vi "VP_RT_standard.vi"() -> ()   [LabVIEW 2015] (continued)
      }
      frame True {
        n40 = shared-variable ".\\Interloop communication.lvlib\\System command"(Command_Enum."Stop System" ("System command")) -> (error out=w66:errorcluster)  [unwired: 1 in]
        n41 = shared-variable ".\\Interloop communication.lvlib\\New Command"(TRUE ("New Command"), error in=w66) -> ()  [unwired: 1 out]
      }
    }
    n42 = Wait Until Next ms Multiple(millisecond multiple=u32 100) -> ()  [unwired: 1 out]
    "Command Loop Iterations" <- w20
  }
  n43 = timed-loop {
    timing: w9 -> [_]
    timing-out: [_] -> w8
    shift-right: [w74] -> _
    shift-left: w4 -> [w71]
    shift-right: [w83] -> _
    shift-left: w2 -> [w75]
    shift-right: [w82] -> _
    shift-left: w1 -> [w76]
    shift-right: [w78] -> _
    shift-left: w3 -> [w79]
    i -> [w80]
    stop <- w85 stop-if-true
    # "Main Loop"
    n44 = node-c288() -> ()  [unwired: 1 in, 1 out]
    n45 = local read "Snake Scan Reference FPGA or EPICS"() -> (w73:enum16{"FPGA Snake Scan", "EPICS Snake Scan"})
    n46 = Format Into String(format string="%s", w71) -> (resulting string=w70:string)  [unwired: 2 in, 1 out]
    n47 = shared-variable "RT CompactRIO Target\\RT_EPICS_Shared_Variables.lvlib\\2iddVELO:VP:RT_State"(w70) -> ()  [unwired: 1 in, 1 out]
    n48 = case shown="\"End Scan\"" w71 {
      tunnel: [w92 w102 w185 w272 w308 w423 w456 w469 w492 w533 w554 w624 w639 w651] -> w84
      tunnel: [FALSE ("Stop") FALSE ("Stop") FALSE ("Stop") FALSE ("Stop") FALSE ("Stop") FALSE ("Stop") FALSE ("Stop") FALSE ("Stop") _ FALSE ("Stop") FALSE ("Stop") FALSE ("Stop") FALSE ("Stop") TRUE ("Stop")] -> w85
      tunnel: [w95 w116 w184 w274 w306 w422 w455 w471 w483 w516 w580 w619 w634 w648] -> w83
      tunnel: [w87 w110 w183 w268 w305 w421 w454 w462 w482 w520 w578 w622 w633 w653] -> w82
      tunnel: w76 -> [w93 w113 w187 w269 w315 w425 w457 w472 w490 w518 w595 w614 w637 w657]
      tunnel: w75 -> [w94 w116 w186 w274 w316 w426 w458 w473 w491 w517 w581 w616 w643 w658]
      tunnel: w79 -> [w92 w102 w185 _ w308 w423 w456 w469 w492 w533 w555 w624 w639 _]
      tunnel: [i64 0 i64 0 i64 0 i64 50 i64 0 i64 0 i64 0 i64 0 i64 0 i64 250 w534 i64 0 i64 0 i64 0] -> w77
      tunnel: w73 -> [_ _ _ _ w302 w418 _ _ _ _ _ _ _ _]
      frame "Initialization", Default {
        n49 = xnode "Invoke Method"("FPGA VI Reference In"=w94, "error in"=w93, "Requested Depth"="Requested Depth") -> ("FPGA VI Reference Out"=w97:refnum<k20>, "error out"=w96:errorcluster, "Actual Depth"=→"Actual Depth":u32)
        n50 = xnode "Read/Write Control"("FPGA VI Reference In"=w97, "error in"=w96, "Datalog Time Period (uSec)"="Datalog Time Period (uSec)", "Datalog Cases"="Datalog Cases") -> ("FPGA VI Reference Out"=w89:refnum<k20>, "error out"=w88:errorcluster)
        n51 = xnode "Read/Write Control"("FPGA VI Reference In"=w89, "error in"=w88) -> ("FPGA VI Reference Out"=w95:refnum<k20>, "error out"=w87:errorcluster, "Wait error"=w86:errorcluster)
        "FPGA wait error" <- w86
        n52 = shared-variable ".\\Interloop communication.lvlib\\FPGA startup error"(w86) -> ()  [unwired: 1 in, 1 out]
      }
      frame "Import Controller coeffs" {
        n53 = call "Read_coeff.vi"("error in (no error)"=w113, "sos gain SF controller file path"="file path sos gain SF Controller_xz1", "sos coeff file path"="file path soscoeff_xz1") -> ("b02(2)"=→"b02(2) xz1c":fxp<+/-,64,9>[], "b01(2)"=→"b01(2) xz1c":fxp<+/-,64,9>[], "-a02(2)"=→"-a02(2) xz1c":fxp<+/-,64,9>[], "-a01(2)"=→"-a01(2) xz1c":fxp<+/-,64,9>[], "error out"=w112:errorcluster, "sos gain SF Controller"=→"sos gain SF Controller xz1c":fxp<+/-,42,9>)  [unwired: 3 in]
        n54 = call "Read_coeff.vi"("error in (no error)"=w113, "sos gain SF controller file path"="file path sos gain SF Controller_xx1", "sos coeff file path"="file path soscoeff_xx1") -> ("b02(2)"=→"b02(2) xx1c":fxp<+/-,64,9>[], "b01(2)"=→"b01(2) xx1c":fxp<+/-,64,9>[], "-a02(2)"=→"-a02(2) xx1c":fxp<+/-,64,9>[], "-a01(2)"=→"-a01(2) xx1c":fxp<+/-,64,9>[], "error out"=w105:errorcluster, "sos gain SF Controller"=→"sos gain SF Controller xx1c":fxp<+/-,42,9>)  [unwired: 3 in]
        n55 = call "Read_coeff.vi"("error in (no error)"=w113, "sos gain SF controller file path"="file path sos gain SF Controller_xy1", "sos coeff file path"="file path soscoeff_xy1") -> ("b02(2)"=→"b02(2) xy1c":fxp<+/-,64,9>[], "b01(2)"=→"b01(2) xy1c":fxp<+/-,64,9>[], "-a02(2)"=→"-a02(2) xy1c":fxp<+/-,64,9>[], "-a01(2)"=→"-a01(2) xy1c":fxp<+/-,64,9>[], "error out"=w108:errorcluster, "sos gain SF Controller"=→"sos gain SF Controller xy1c":fxp<+/-,42,9>)  [unwired: 3 in]
        n56 = call "Read_coeff.vi"("error in (no error)"=w112, "sos gain SF controller file path"="file path sos gain SF Controller_yz1", "sos coeff file path"="file path soscoeff_yz1") -> ("b02(2)"=→"b02(2) yz1c":fxp<+/-,64,9>[], "b01(2)"=→"b01(2) yz1c":fxp<+/-,64,9>[], "-a02(2)"=→"-a02(2) yz1c":fxp<+/-,64,9>[], "-a01(2)"=→"-a01(2) yz1c":fxp<+/-,64,9>[], "error out"=w111:errorcluster, "sos gain SF Controller"=→"sos gain SF Controller yz1c":fxp<+/-,42,9>)  [unwired: 3 in]
        n57 = call "Read_coeff.vi"("error in (no error)"=w108, "sos gain SF controller file path"="file path sos gain SF Controller_yy1", "sos coeff file path"="file path soscoeff_yy1") -> ("b02(2)"=→"b02(2) yy1c":fxp<+/-,64,9>[], "b01(2)"=→"b01(2) yy1c":fxp<+/-,64,9>[], "-a02(2)"=→"-a02(2) yy1c":fxp<+/-,64,9>[], "-a01(2)"=→"-a01(2) yy1c":fxp<+/-,64,9>[], "error out"=w107:errorcluster, "sos gain SF Controller"=→"sos gain SF Controller yy1c":fxp<+/-,42,9>)  [unwired: 3 in]
        n58 = call "Read_coeff.vi"("error in (no error)"=w105, "sos gain SF controller file path"="file path sos gain SF Controller_yx1", "sos coeff file path"="file path soscoeff_yx1") -> ("b02(2)"=→"b02(2) yx1c":fxp<+/-,64,9>[], "b01(2)"=→"b01(2) yx1c":fxp<+/-,64,9>[], "-a02(2)"=→"-a02(2) yx1c":fxp<+/-,64,9>[], "-a01(2)"=→"-a01(2) yx1c":fxp<+/-,64,9>[], "error out"=w104:errorcluster, "sos gain SF Controller"=→"sos gain SF Controller yx1c":fxp<+/-,42,9>)  [unwired: 3 in]
        n59 = call "Read_coeff.vi"("error in (no error)"=w111, "sos gain SF controller file path"="file path sos gain SF Controller_zz1", "sos coeff file path"="file path soscoeff_zz1") -> ("b02(2)"=→"b02(2) zz1c":fxp<+/-,64,9>[], "b01(2)"=→"b01(2) zz1c":fxp<+/-,64,9>[], "-a02(2)"=→"-a02(2) zz1c":fxp<+/-,64,9>[], "-a01(2)"=→"-a01(2) zz1c":fxp<+/-,64,9>[], "error out"=w109:errorcluster, "sos gain SF Controller"=→"sos gain SF Controller zz1c":fxp<+/-,42,9>)  [unwired: 3 in]
        n60 = call "Read_coeff.vi"("error in (no error)"=w104, "sos gain SF controller file path"="file path sos gain SF Controller_zx1", "sos coeff file path"="file path soscoeff_zx1") -> ("b02(2)"=→"b02(2) zx1c":fxp<+/-,64,9>[], "b01(2)"=→"b01(2) zx1c":fxp<+/-,64,9>[], "-a02(2)"=→"-a02(2) zx1c":fxp<+/-,64,9>[], "-a01(2)"=→"-a01(2) zx1c":fxp<+/-,64,9>[], "error out"=w103:errorcluster, "sos gain SF Controller"=→"sos gain SF Controller zx1c":fxp<+/-,42,9>)  [unwired: 3 in]
        n61 = call "Read_coeff.vi"("error in (no error)"=w107, "sos gain SF controller file path"="file path sos gain SF Controller_zy1", "sos coeff file path"="file path soscoeff_zy1") -> ("b02(2)"=→"b02(2) zy1c":fxp<+/-,64,9>[], "b01(2)"=→"b01(2) zy1c":fxp<+/-,64,9>[], "-a02(2)"=→"-a02(2) zy1c":fxp<+/-,64,9>[], "-a01(2)"=→"-a01(2) zy1c":fxp<+/-,64,9>[], "error out"=w106:errorcluster, "sos gain SF Controller"=→"sos gain SF Controller zy1c":fxp<+/-,42,9>)  [unwired: 3 in]
        n62 = Merge Errors(w113, w103, w106, w109) -> (w110:errorcluster)
        "Coeff file import error" <- w110
      }
      frame "Update Controller Info" {
        n63 = local read "sos gain SF Controller yy1c"() -> (w246:fxp<+/-,42,9>)
        n64 = local read "sos gain SF Controller yz1c"() -> (w195:fxp<+/-,42,9>)
        n65 = local read "sos gain SF Controller yx1c"() -> (w234:fxp<+/-,42,9>)
        n66 = local read "sos gain SF Controller xy1c"() -> (w220:fxp<+/-,42,9>)
        n67 = local read "sos gain SF Controller zy1c"() -> (w225:fxp<+/-,42,9>)
        n68 = local read "sos gain SF Controller xz1c"() -> (w209:fxp<+/-,42,9>)
        n69 = local read "sos gain SF Controller xx1c"() -> (w251:fxp<+/-,42,9>)
        n70 = local read "sos gain SF Controller zz1c"() -> (w244:fxp<+/-,42,9>)
        n71 = local read "sos gain SF Controller zx1c"() -> (w230:fxp<+/-,42,9>)
        n72 = local read "-a01(2) yy1c"() -> (w250:fxp<+/-,64,9>[])
        n73 = local read "-a02(2) yy1c"() -> (w249:fxp<+/-,64,9>[])
        n74 = local read "-a01(2) yz1c"() -> (w214:fxp<+/-,64,9>[])
        n75 = local read "-a02(2) yz1c"() -> (w215:fxp<+/-,64,9>[])
        n76 = local read "-a01(2) yx1c"() -> (w235:fxp<+/-,64,9>[])
        n77 = local read "-a02(2) yx1c"() -> (w231:fxp<+/-,64,9>[])
        n78 = local read "-a01(2) xy1c"() -> (w216:fxp<+/-,64,9>[])
        n79 = local read "-a02(2) xy1c"() -> (w217:fxp<+/-,64,9>[])
        n80 = local read "-a01(2) zy1c"() -> (w221:fxp<+/-,64,9>[])
        n81 = local read "-a02(2) zy1c"() -> (w222:fxp<+/-,64,9>[])
        n82 = local read "-a01(2) xz1c"() -> (w213:fxp<+/-,64,9>[])
        n83 = local read "-a02(2) xz1c"() -> (w212:fxp<+/-,64,9>[])
        n84 = local read "-a01(2) xx1c"() -> (w255:fxp<+/-,64,9>[])
        n85 = local read "-a02(2) xx1c"() -> (w254:fxp<+/-,64,9>[])
        n86 = local read "-a01(2) zz1c"() -> (w245:fxp<+/-,64,9>[])
        n87 = local read "-a02(2) zz1c"() -> (w241:fxp<+/-,64,9>[])
        n88 = local read "-a01(2) zx1c"() -> (w226:fxp<+/-,64,9>[])
        n89 = local read "-a02(2) zx1c"() -> (w227:fxp<+/-,64,9>[])
        n90 = local read "b01(2) yy1c"() -> (w248:fxp<+/-,64,9>[])
        n91 = local read "b02(2) yy1c"() -> (w247:fxp<+/-,64,9>[])
        n92 = local read "b01(2) yz1c"() -> (w189:fxp<+/-,64,9>[])
        n93 = local read "b02(2) yz1c"() -> (w188:fxp<+/-,64,9>[])
        n94 = local read "b01(2) yx1c"() -> (w232:fxp<+/-,64,9>[])
        n95 = local read "b02(2) yx1c"() -> (w233:fxp<+/-,64,9>[])
        n96 = local read "b01(2) xy1c"() -> (w218:fxp<+/-,64,9>[])
        n97 = local read "b02(2) xy1c"() -> (w219:fxp<+/-,64,9>[])
        n98 = local read "b01(2) zy1c"() -> (w223:fxp<+/-,64,9>[])
        n99 = local read "b02(2) zy1c"() -> (w224:fxp<+/-,64,9>[])
        n100 = local read "b01(2) xz1c"() -> (w211:fxp<+/-,64,9>[])
        n101 = local read "b02(2) xz1c"() -> (w210:fxp<+/-,64,9>[])
        n102 = local read "b01(2) xx1c"() -> (w253:fxp<+/-,64,9>[])
        n103 = local read "b02(2) xx1c"() -> (w252:fxp<+/-,64,9>[])
        n104 = local read "b01(2) zz1c"() -> (w242:fxp<+/-,64,9>[])
        n105 = local read "b02(2) zz1c"() -> (w243:fxp<+/-,64,9>[])
        n106 = local read "b01(2) zx1c"() -> (w228:fxp<+/-,64,9>[])
        n107 = local read "b02(2) zx1c"() -> (w229:fxp<+/-,64,9>[])
        n108 = Or(x="Optics Z Reset", y="Reset All") -> (x .or. y?=w208:bool)
        n109 = Or(x="Sample Z Reset", y="Reset All") -> (x .or. y?=w205:bool)
        n110 = Or(x="Optics X Reset", y="Reset All") -> (x .or. y?=w239:bool)
        n111 = Or(x="Optics Y Reset", y="Reset All") -> (x .or. y?=w237:bool)
        n112 = Or(x="Sample X Reset", y="Reset All") -> (x .or. y?=w207:bool)
        n113 = Or(x="Sample Y Reset", y="Reset All") -> (x .or. y?=w206:bool)
        n114 = xnode "Read/Write Control"("FPGA VI Reference In"=w186, "error in"=w187, "Wait timer (ms)"="FPGA Wait Timer (ms)", "Controller Time Period (uSec)"="Controller Time Period (uSec)", "Controller Output Time Period (uSec)"="Controller Output Time Period (uSec)", "System Loop Type"="System Loop Type", "Controller Output Upper Limit"="Controller Output Upper Limit", "Controller Output Lower Limit"="Controller Output Lower Limit", "X-Stage nm to V Scaling"="X-Stage nm to V Scaling", "X-Stage Scaling Direction"="X-Stage Scaling Direction", "Y-Stage nm to V Scaling"="Y-Stage nm to V Scaling", "Z-Stage nm to V Scaling"="Z-Stage nm to V Scaling", "Plant Output Time Period (uSec)"="Plant Output Time Period (uSec)", "Reset Optics X"=w239, "Reset Optics Y"=w237, "Reset Optics Z"=w208, "Reset Sample X"=w207, "Reset Sample Y"=w206, "Reset Sample Z"=w205, "Optics X Stage Resolution (nm)"="Optics X Stage Resolution (nm)", "Optics Y Stage Resolution (nm)"="Optics Y Stage Resolution (nm)", "Optics Z Stage Resolution (nm)"="Optics Z Stage Resolution (nm)", "Sample X Stage Resolution (nm)"="Sample X Stage Resolution (nm)", "Sample Y Stage Resolution (nm)"="Sample Y Stage Resolution (nm)", "Sample Z Stage Resolution (nm)"="Sample Z Stage Resolution (nm)", "Scaling mV to V"="Scaling mV to V", "-a01(2) xx1"=w255, "-a02(2) xx1"=w254, "b01(2) xx1"=w253, "b02(2) xx1"=w252, "sos gain SF Controller xx1"=w251, "-a01(2) yy1"=w250, "-a02(2) yy1"=w249, "b01(2) yy1"=w248, "b02(2) yy1"=w247, "sos gain SF Controller yy1"=w246, "-a01(2) zz1"=w245, "-a02(2) zz1"=w241, "b01(2) zz1"=w242, "b02(2) zz1"=w243, "sos gain SF Controller zz1"=w244, "-a01(2) yx1"=w235, "-a02(2) yx1"=w231, "b01(2) yx1"=w232, "b02(2) yx1"=w233, "sos gain SF Controller yx1"=w234, "-a01(2) zx1"=w226, "-a02(2) zx1"=w227, "b01(2) zx1"=w228, "b02(2) zx1"=w229, "sos gain SF Controller zx1"=w230, "-a01(2) xy1"=w216, "-a02(2) xy1"=w217, "b01(2) xy1"=w218, "b02(2) xy1"=w219, "sos gain SF Controller xy1"=w220, "-a01(2) zy1"=w221, "-a02(2) zy1"=w222, "b01(2) zy1"=w223, "b02(2) zy1"=w224, "sos gain SF Controller zy1"=w225, "-a01(2) xz1"=w213, "-a02(2) xz1"=w212, "b01(2) xz1"=w211, "b02(2) xz1"=w210, "sos gain SF Controller xz1"=w209, "-a01(2) yz1"=w214, "-a02(2) yz1"=w215, "b01(2) yz1"=w189, "b02(2) yz1"=w188, "sos gain SF Controller yz1"=w195, "Analog Input Time Period (uSec)"="Analog Input Time Period (uSec)", "Optics and or Sample Stage"="Optics and or Sample Stage", "Y-Stage Scaling Direction"="Y-Stage Scaling Direction", "Z-Stage Scaling Direction"="Z-Stage Scaling Direction") -> ("FPGA VI Reference Out"=w184:refnum<k20>, "error out"=w183:errorcluster)
      }
      frame "Wait" {
        n115 = shared-variable ".\\Interloop communication.lvlib\\New Command"() -> (w273:bool, error out=w271:errorcluster)  [unwired: 1 in]
        n116 = case shown="True" w273 {
          tunnel: [w276 w277] -> w272
          tunnel: w271 -> [_ w281]
          tunnel: w269 -> [w275 w279]
          tunnel: [w275 w278] -> w268
          frame False {
            w276 = T10[] [enum."Wait"] items=["Initialization", "Import Controller coeffs", "Update Controller Info", "Wait", "Update Reference Info", "Update Detector Trigger Info", "Update Datalog Info", "Check FPGA Status", "Pre-Scan", "Start Scan", "Scanning", "End Scan", "Restart FPGA", "Stop FPGA"]
          }
          frame True {
            n117 = shared-variable ".\\Interloop communication.lvlib\\System command"() -> (w280:T7)  [unwired: 1 in, 1 out]
            "Last Command Executed" <- w280
            n118 = case shown="\"Stop System\"" w280 {
              tunnel: [w285 w288 w291 w294 w297 w301] -> w277
              tunnel: w279 -> [w284 w287 w290 w293 w296 w300]
              tunnel: [w283 w286 w289 w292 w295 w299] -> w278
              frame "Re-Initialize ", Default {
                w285 = T10[] [enum."Initialization", enum."Import Controller coeffs", enum."Update Controller Info", enum."Wait"] items=["Initialization", "Import Controller coeffs", "Update Controller Info", "Wait", "Update Reference Info", "Update Detector Trigger Info", "Update Datalog Info", "Check FPGA Status", "Pre-Scan", "Start Scan", "Scanning", "End Scan", "Restart FPGA", "Stop FPGA"]
                n119 = call <vilib>:"Clear Errors.vi"("error in (no error)"=w284) -> ("error out"=w283:errorcluster)  [unwired: 5 in, 1 out]
              }
              frame "Update Scan Settings" {
                w288 = T10[] [enum."Update Reference Info", enum."Update Detector Trigger Info", enum."Update Datalog Info", enum."Wait"] items=["Initialization", "Import Controller coeffs", "Update Controller Info", "Wait", "Update Reference Info", "Update Detector Trigger Info", "Update Datalog Info", "Check FPGA Status", "Pre-Scan", "Start Scan", "Scanning", "End Scan", "Restart FPGA", "Stop FPGA"]
                n120 = call <vilib>:"Clear Errors.vi"("error in (no error)"=w287) -> ("error out"=w286:errorcluster)  [unwired: 5 in, 1 out]
              }
              frame "Scan" {
                w291 = T10[] [enum."Update Reference Info", enum."Update Detector Trigger Info", enum."Update Datalog Info", enum."Pre-Scan", enum."Start Scan", enum."Scanning", enum."End Scan", enum."Wait"] items=["Initialization", "Import Controller coeffs", "Update Controller Info", "Wait", "Update Reference Info", "Update Detector Trigger Info", "Update Datalog Info", "Check FPGA Status", "Pre-Scan", "Start Scan", "Scanning", "End Scan", "Restart FPGA", "Stop FPGA"]
                n121 = call <vilib>:"Clear Errors.vi"("error in (no error)"=w290) -> ("error out"=w289:errorcluster)  [unwired: 5 in, 1 out]
              }
              frame "Stop Scan" {
                w294 = T10[] [enum."End Scan", enum."Wait"] items=["Initialization", "Import Controller coeffs", "Update Controller Info", "Wait", "Update Reference Info", "Update Detector Trigger Info", "Update Datalog Info", "Check FPGA Status", "Pre-Scan", "Start Scan", "Scanning", "End Scan", "Restart FPGA", "Stop FPGA"]
                n122 = call <vilib>:"Clear Errors.vi"("error in (no error)"=w293) -> ("error out"=w292:errorcluster)  [unwired: 5 in, 1 out]
              }
              frame "Restart FPGA" {
                w297 = T10[] [enum."Restart FPGA", enum."Initialization", enum."Import Controller coeffs", enum."Update Controller Info", enum."Wait"] items=["Initialization", "Import Controller coeffs", "Update Controller Info", "Wait", "Update Reference Info", "Update Detector Trigger Info", "Update Datalog Info", "Check FPGA Status", "Pre-Scan", "Start Scan", "Scanning", "End Scan", "Restart FPGA", "Stop FPGA"]
                n123 = call <vilib>:"Clear Errors.vi"("error in (no error)"=w296) -> ("error out"=w295:errorcluster)  [unwired: 5 in, 1 out]
              }
              frame "Stop System" {
                w301 = T10[] [enum."Stop FPGA"] items=["Initialization", "Import Controller coeffs", "Update Controller Info", "Wait", "Update Reference Info", "Update Detector Trigger Info", "Update Datalog Info", "Check FPGA Status", "Pre-Scan", "Start Scan", "Scanning", "End Scan", "Restart FPGA", "Stop FPGA"]
                n124 = call <vilib>:"Clear Errors.vi"("error in (no error)"=w300) -> ("error out"=w299:errorcluster)  [unwired: 5 in, 1 out]
                n125 = local write "Stop System (Careful!!)"(TRUE ("Stop")) -> ()
              }
            }
            n126 = shared-variable ".\\Interloop communication.lvlib\\New Command"(FALSE ("New Command"), error in=w281) -> ()  [unwired: 1 out]
          }
        }
      }
      frame "Update Reference Info" {
        w368 = errorcluster {"status"=FALSE, "code"=0, "source"=""}  # error in (no error)
        w371 = errorcluster {"status"=FALSE, "code"=0, "source"=""}  # error in (no error)
        w385 = errorcluster {"status"=FALSE, "code"=0, "source"=""}  # error in (no error)
        w364 = 40000000.0  # FPGA clock rate (Hz)
        n127 = local read "Measured Z Reference Time Period (Ticks)"() -> (w307:u32)
        n128 = case shown="\"EPICS Snake Scan\"" w302 {
          tunnel: ["X Ramp Start (nm)" w401] -> w323
          tunnel: ["X Ramp End (nm)" w400] -> w322
          tunnel: ["Y Ramp Start (nm)" w399] -> w321
          tunnel: ["Y Ramp End (nm)" w398] -> w320
          tunnel: ["Y Step Size (nm)" w402] -> w319
          tunnel: ["X Step Size (nm)" w405] -> w318
          tunnel: [w393 w403] -> w317
          tunnel: ["Y Step Size (nm)" w402] -> w314
          tunnel: ["X Ramp Start (nm)" w401] -> w313
          tunnel: ["X Ramp End (nm)" w400] -> w312
          tunnel: ["Y Ramp Start (nm)" w399] -> w311
          tunnel: ["Y Ramp End (nm)" w398] -> w310
          frame "FPGA Snake Scan", Default {
            n129 = local read "DT Frequency (Hz)"() -> (w393:dbl)
          }
          frame "EPICS Snake Scan" {
            w404 = fxp<+/-,16,16> 0.0 ("fixed-point type")
            n130 = shared-variable "RT CompactRIO Target\\RT_EPICS_Shared_Variables.lvlib\\2iddVELO:VP:Trigger_Freq_Hz"() -> (w403:dbl)  [unwired: 1 in, 1 out]
            "2iddVELO:VP:Trigger_Freq_Hz" <- w403
            n131 = shared-variable "RT CompactRIO Target\\RT_EPICS_Shared_Variables.lvlib\\2iddVELO:VP:Y_Step_Size_nm"() -> (w407:dbl)  [unwired: 1 in, 1 out]
            "2iddVELO:VP:Y_Step_Size_nm" <- w407
            n132 = shared-variable "RT CompactRIO Target\\RT_EPICS_Shared_Variables.lvlib\\2iddVELO:VP:X_Step_Size_nm"() -> (w406:dbl)  [unwired: 1 in, 1 out]
            "2iddVELO:VP:X_Step_Size_nm" <- w406
            n133 = shared-variable "RT CompactRIO Target\\RT_EPICS_Shared_Variables.lvlib\\2iddVELO:VP:Y_Start_nm"() -> (w408:dbl)  [unwired: 1 in, 1 out]
            n134 = shared-variable "RT CompactRIO Target\\RT_EPICS_Shared_Variables.lvlib\\2iddVELO:VP:Y_End_nm"() -> (w397:dbl)  [unwired: 1 in, 1 out]
            n135 = shared-variable "RT CompactRIO Target\\RT_EPICS_Shared_Variables.lvlib\\2iddVELO:VP:X_Start_nm"() -> (w410:dbl)  [unwired: 1 in, 1 out]
            "2iddVELO:VP:X_Start_nm" <- w410
            n136 = shared-variable "RT CompactRIO Target\\RT_EPICS_Shared_Variables.lvlib\\2iddVELO:VP:X_End_nm"() -> (w409:dbl)  [unwired: 1 in, 1 out]
            "2iddVELO:VP:X_End_nm" <- w409
            n137 = Negate(x=w397) -> (-x=w396:dbl)
            "2iddVELO:VP:Y_End_nm" <- w396
            n138 = Negate(x=w408) -> (-x=w395:dbl)
            "2iddVELO:VP:Y_Start_nm" <- w395
            n139 = To Fixed-Point(fixed-point type=w404, number=w410) -> (fixed-point=w401:fxp<+/-,16,16>)
            n140 = To Fixed-Point(fixed-point type=w404, number=w409) -> (fixed-point=w400:fxp<+/-,16,16>)
            n141 = To Fixed-Point(fixed-point type=w404, number=w395) -> (fixed-point=w399:fxp<+/-,16,16>)
            n142 = To Fixed-Point(fixed-point type=w404, number=w396) -> (fixed-point=w398:fxp<+/-,16,16>)
            n143 = To Fixed-Point(fixed-point type=w404, number=w407) -> (fixed-point=w402:fxp<+/-,16,16>)
            n144 = To Fixed-Point(fixed-point type=w404, number=w406) -> (fixed-point=w405:fxp<+/-,16,16>)
          }
        }
        n145 = local read "Y Ramp Period (usec)"() -> (w325:fxp<+,24,24>)
        n146 = shared-variable ".\\Interloop communication.lvlib\\Fly Scan Flag"() -> (w309:bool)  [unwired: 1 in, 1 out]
        n147 = case shown="\"Sawtooth Wave\"" "Z Reference Wave Selection" {
          tunnel: "Z frequency (Hz)" -> [w411 w412 w414 w416 w417]
          tunnel: [w411 w412 w413 w416 w417] -> w346
          tunnel: w307 -> [_ _ w415 _ _]
          frame "Constant", Default {
          }
          frame "Sine Wave" {
          }
          frame "Sawtooth Wave" {
            n148 = Multiply(x=w415, y=w414) -> (x*y=w413:dbl)
          }
          frame "Square Wave" {
          }
          frame "Filtered White Noise" {
          }
        }
        n149 = call <vilib>:"Normalize Signal Generation Parameters.vi"("frequency (Hz)"="X frequency (Hz)", "FPGA clock rate (Hz)"=w364, "phase offset (deg)"="X phase offset (deg)", "error in (no error)"=w385) -> ("frequency (periods/tick)"=w384:fxp<+,32,0>, "phase offset (periods)"=w374:fxp<+,32,0>, "error out"=→"error out (Sig Gen)":errorcluster)  [unwired: 6 in, 3 out]
        "X frequency (periods/tick)" <- w384
        "X phase offset (periods)" <- w374
        n150 = call <vilib>:"Normalize Signal Generation Parameters.vi"("frequency (Hz)"="Y frequency (Hz)", "FPGA clock rate (Hz)"=w364, "phase offset (deg)"="Y phase offset (deg)", "error in (no error)"=w371) -> ("frequency (periods/tick)"=w367:fxp<+,32,0>, "phase offset (periods)"=w366:fxp<+,32,0>, "error out"=→"error out (Sig Gen) 2":errorcluster)  [unwired: 6 in, 3 out]
        "Y frequency (periods/tick)" <- w367
        "Y phase offset (periods)" <- w366
        n151 = call <vilib>:"Normalize Signal Generation Parameters.vi"("frequency (Hz)"=w346, "FPGA clock rate (Hz)"=w364, "phase offset (deg)"="Z phase offset (deg)", "error in (no error)"=w368) -> ("frequency (periods/tick)"=w365:fxp<+,32,0>, "phase offset (periods)"=w357:fxp<+,32,0>, "error out"=→"error out (Sig Gen) 3":errorcluster)  [unwired: 6 in, 3 out]
        "Z frequency (periods/tick)" <- w365
        "Z phase offset (periods)" <- w357
        n152 = local read "X Ramp Period (usec)"() -> (w324:fxp<+,24,24>)
        n153 = xnode "Read/Write Control"("FPGA VI Reference In"=w316, "error in"=w315, "X Reference Time Period (uSec)"="X Reference Time Period (uSec)", "Y Reference Time Period (uSec)"="Y Reference Time Period (uSec)", "Z Reference Time Period (uSec)"="Z Reference Time Period (uSec)", "X Reference Wave Selection"="X Reference Wave Selection", "Y Reference Wave Selection"="Y Reference Wave Selection", "Z Reference Wave Selection"="Z Reference Wave Selection", "X Reference Reset"="X Reference Reset", "Y Reference Reset"="Y Reference Reset", "Z Reference Reset"="Z Reference Reset", "X Reference Amplitude (nm)"="X Reference Amplitude (nm)", "Y Reference Amplitude (nm)"="Y Reference Amplitude (nm)", "Z Reference Amplitude (nm)"="Z Reference Amplitude (nm)", "X Frequency (periods/tick)"=w384, "X Phase Offset (periods)"=w374, "Y Frequency (periods/tick)"=w367, "Y Phase Offset (periods)"=w366, "Z Frequency (periods/tick)"=w365, "Z Phase Offset (periods)"=w357, "X Reference DC Offset (nm)"="X Reference DC Offset (nm)", "Y Reference DC Offset (nm)"="Y Reference DC Offset (nm)", "Z Reference DC Offset (nm)"="Z Reference DC Offset (nm)", "X White Noise Amplitude"="X White Noise Amplitude", "X White Noise Seed"="X White Noise Seed", "Y White Noise Amplitude"="Y White Noise Amplitude", "Y White Noise Seed"="Y White Noise Seed", "Z White Noise Amplitude"="Z White Noise Amplitude", "Z White Noise Seed"="Z White Noise Seed", "Mod 3 AI0 V to nm Scaling"="Mod 3 AI0 V to nm Scaling", "Mod 3 AI1 V to nm Scaling"="Mod 3 AI1 V to nm Scaling", "Mod 3 AI2 V to nm Scaling"="Mod 3 AI2 V to nm Scaling", "X Ramp Period (usec)"=w324, "X Ramp Start (nm)"=w323, "X Ramp End (nm)"=w322, "X Start Marker (nm)"="X Start Marker (nm)", "Fly Scan"=w309, "Y Ramp Period (usec)"=w325, "Y Ramp Start (nm)"=w321, "Y Ramp End (nm)"=w320, "Y Ramp Drop Size (nm)"=w319, "Y Start Marker (nm)"="Y Start Marker (nm)") -> ("FPGA VI Reference Out"=w306:refnum<k20>, "error out"=w305:errorcluster)
        n154 = Subtract(x=w311, y=w310) -> (x-y=w341:fxp<+/-,17,17>)
        n155 = Subtract(x=w313, y=w312) -> (x-y=w339:fxp<+/-,17,17>)
        n156 = Absolute Value(x=w341) -> (abs(x)=w332:fxp<+,16,16>)
        n157 = Absolute Value(x=w339) -> (abs(x)=w338:fxp<+,16,16>)
        n158 = Divide(x=w338, y=w318) -> (x/y=w336:fxp<+/-,33,17>)
        "# of Points per Line" <- w336
        n159 = Divide(x=w336, y=w317) -> (x/y=w328:dbl)
        "sec per line" <- w328
        n160 = Divide(x=w332, y=w314) -> (x/y=w333:fxp<+/-,33,17>)
        n161 = Add(x=w333, y=fxp<+,16,16> 1.0) -> (x+y=w327:fxp<+/-,34,18>)
        "# of Hor Lines" <- w327
        n162 = Multiply(x=w328, y=1000000.0) -> (x*y=w331:dbl)
        "X Ramp Period DBL (usec)" <- w331
        n163 = Reciprocal(x=w328) -> (1/x=→"line per sec (Hz)":dbl)
        n164 = To Fixed-Point(fixed-point type=fxp<+,24,24> 0.0, number=w331) -> (fixed-point=→"X Ramp Period (usec)" →"Y Ramp Period (usec)":fxp<+,24,24>)
        n165 = Multiply(x=w328, y=w327) -> (x*y=→"Total Scan Time (sec)":dbl)
        n166 = Multiply(x=w327, y=w336) -> (x*y=→"# Total Trigger Points":fxp<+/-,64,34>)
      }
      frame "Update Detector Trigger Info" {
        w432 = 40000000.0  # FPGA clock rate (Hz)
        w434 = errorcluster {"status"=FALSE, "code"=0, "source"=""}  # error in (no error)
        n167 = case shown="\"EPICS Snake Scan\"" w418 {
          tunnel: ["DT Frequency (Hz)" w451] -> w433
          tunnel: ["DT duty cycle (%)" w450] -> w427
          frame "FPGA Snake Scan", Default {
          }
          frame "EPICS Snake Scan" {
            n168 = shared-variable "RT CompactRIO Target\\RT_EPICS_Shared_Variables.lvlib\\2iddVELO:VP:Trig_DutyCycle_Per"() -> (w450:dbl)  [unwired: 1 in, 1 out]
            "2iddVELO:VP:Trig_DutyCycle_Per" <- w450
            n169 = shared-variable "RT CompactRIO Target\\RT_EPICS_Shared_Variables.lvlib\\2iddVELO:VP:Trigger_Freq_Hz"() -> (w451:dbl)  [unwired: 1 in, 1 out]
          }
        }
        "Trigger Frequency (Hz)" <- w433
        "Trigger Duty Cycle (%)" <- w427
        n170 = call <vilib>:"Normalize Signal Generation Parameters.vi"("frequency (Hz)"=w433, "FPGA clock rate (Hz)"=w432, "phase offset (deg)"="DT phase offset (deg)", "duty cycle (%)"=w427, "error in (no error)"=w434) -> ("frequency (periods/tick)"=w430:fxp<+,32,0>, "phase offset (periods)"=w429:fxp<+,32,0>, "duty cycle (periods)"=w428:fxp<+,32,0>, "error out"=→"error out (Sig Gen) 4":errorcluster)  [unwired: 5 in, 2 out]
        "DT Frequency (periods/tick)" <- w430
        "DT Phase Offset (periods)" <- w429
        "DT Duty Cycle (periods)" <- w428
        n171 = xnode "Read/Write Control"("FPGA VI Reference In"=w426, "error in"=w425, "Detector Trigger Time Period (uSec)"="Detector Trigger Time Period (uSec)", "Trigger Generation Time Period (uSec)"="Trigger Generation Time Period (uSec)", "Detector Trigger Lower Limit (V)"="Detector Trigger Lower Limit (V)", "Detector Trigger Upper Limit (V)"="Detector Trigger Upper Limit (V)", "Trigger High Period (usec)"="Trigger High Period (usec)", "Trigger Low Period (usec)"="Trigger Low Period (usec)", "Trigger High Level (V)"="Trigger High Level (V)", "Trigger Low Level (V)"="Trigger Low Level (V)", "Trigger Wave Generator"="Trigger Wave Generator", "DT Reference Amplitude (V)"="DT Reference Amplitude (V)", "DT Reference DC Offset (V)"="DT Reference DC Offset (V)", "DT Frequency (periods/tick)"=w430, "DT Phase Offset (periods)"=w429, "DT Reset"="DT Reset", "DT Duty Cycle (periods)"=w428, "Data Trigger Time Period (uSec)"="Data Trigger Time Period (uSec)") -> ("FPGA VI Reference Out"=w422:refnum<k20>, "error out"=w421:errorcluster)
      }
      frame "Update Datalog Info" {
        n172 = local read "Datalog Time Period (uSec)"() -> (w461:u32)
        n173 = local read "Datalog Cases"() -> (w460:T2)
        n174 = xnode "Read/Write Control"("FPGA VI Reference In"=w458, "error in"=w457, "Datalog Time Period (uSec)"=w461, "Datalog Cases"=w460, "Timeout FPGA FIFO1"="Timeout FPGA FIFO1") -> ("FPGA VI Reference Out"=w455:refnum<k20>, "error out"=w454:errorcluster)
      }
      frame "Check FPGA Status" {
        n175 = xnode "Read/Write Control"("FPGA VI Reference In"=w473, "error in"=w472) -> ("FPGA VI Reference Out"=w471:refnum<k20>, "error out"=w470:errorcluster, "FPGA error monitor"=w476:errorcluster, "End Run Error"=w475:errorcluster, "FIFO Timed Out?"=→"FIFO Timed Out?":bool, "stop case"=w465:bool, "FIFO Timed Out"=w466:bool)
        "FPGA error monitor" <- w476
        "FPGA end run error" <- w475
        "stop case" <- w465
        "FIFO Timed Out" <- w466
        n176 = case shown="True" w465 {
          tunnel: [errorcluster {"status"=FALSE, "code"=0, "source"=""} ("error constant") errorcluster {"status"=TRUE, "code"=7002, "source"="FPGA stop case encountered"} ("error constant")] -> w463
          frame False {
          }
          frame True {
          }
        }
        n177 = case shown="True" w466 {
          tunnel: [errorcluster {"status"=FALSE, "code"=0, "source"=""} ("error constant") errorcluster {"status"=TRUE, "code"=7001, "source"="FPGA FIFO timed out"} ("error constant")] -> w464
          frame False {
          }
          frame True {
          }
        }
        n178 = Merge Errors(w470, w476, w475, w463, w464) -> (w462:errorcluster)
      }
      frame "Pre-Scan" {
        n179 = flat-sequence {
          tunnel: w491 -> [w498]
          tunnel: w490 -> [w497]
          tunnel: [w494] -> w489
          tunnel: [w493] -> w487
          tunnel: w489 -> [w504]
          tunnel: [w504] -> w488
          tunnel: w487 -> [w503]
          tunnel: [w503] -> w486
          tunnel: w488 -> [w508]
          tunnel: w486 -> [w507]
          tunnel: [w506] -> w485
          tunnel: [w505] -> w484
          tunnel: w485 -> [w515]
          tunnel: w484 -> [w514]
          tunnel: [w511] -> w483
          tunnel: [w510] -> w482
          frame #0 {
            w495 = TRUE
            n180 = xnode "Read/Write Control"("FPGA VI Reference In"=w498, "error in"=w497, "Reset Optics X"=w495, "Reset Optics Y"=w495, "Reset Optics Z"=w495, "Reset Sample X"=w495, "Reset Sample Y"=w495, "Reset Sample Z"=w495, "System Loop Type"=enum16{"Open Loop", "Closed Loop"}."Open Loop", "New FPGA command"=TRUE, "FPGA command"=enum16{"Start Scan", "Shutdown"}."Start Scan", "Fly Scan"=FALSE) -> ("FPGA VI Reference Out"=w494:refnum<k20>, "error out"=w493:errorcluster)
          }
          frame #1 {
            n181 = Wait (ms)(milliseconds to wait="Pre-Scan pause (ms)") -> ()  [unwired: 1 out]
          }
          frame #2 {
            n182 = xnode "Read/Write Control"("FPGA VI Reference In"=w508, "error in"=w507, "stop case"=TRUE) -> ("FPGA VI Reference Out"=w506:refnum<k20>, "error out"=w505:errorcluster)
          }
          frame #3 {
            w512 = FALSE ("Reset Optics X")
            n183 = local read "System Loop Type"() -> (w513:enum16{"Open Loop", "Closed Loop"})
            n184 = xnode "Read/Write Control"("FPGA VI Reference In"=w515, "error in"=w514, "Reset Optics X"=w512, "Reset Optics Y"=w512, "Reset Optics Z"=w512, "Reset Sample X"=w512, "Reset Sample Y"=w512, "Reset Sample Z"=w512, "System Loop Type"=w513) -> ("FPGA VI Reference Out"=w511:refnum<k20>, "error out"=w510:errorcluster)
          }
        }
      }
      frame "Start Scan" {
        n185 = shared-variable ".\\Interloop communication.lvlib\\Base Filename"() -> (w521:string)  [unwired: 1 in, 1 out]
        n186 = String To Path(string="cRIO data dir") -> (path=w522:path)
        "cRIO path" <- w522
        n187 = call "Data_Write.vi"("Destination dir"=w522, "error initialize"=w518, "Base name"=w521, "Command List"=Data_Write_Control."Initialize") -> ("error out"=w519:errorcluster, "Path"=w530:path)  [unwired: 4 in]
        n188 = Strip Path(path=w530) -> (stripped path=→"Output path":path, name=→"Output filename":string)
        n189 = shared-variable ".\\Interloop communication.lvlib\\Fly Scan Flag"() -> (w525:bool)  [unwired: 1 in, 1 out]
        n190 = xnode "Read/Write Control"("FPGA VI Reference In"=w517, "error in"=w519, "New FPGA command"=TRUE, "FPGA command"=enum16{"Start Scan", "Shutdown"}."Start Scan", "Fly Scan"=w525) -> ("FPGA VI Reference Out"=w516:refnum<k20>, "error out"=w520:errorcluster)
        n191 = shared-variable "RT CompactRIO Target\\RT_EPICS_Shared_Variables.lvlib\\2iddVELO:VP:Scanning"(w525) -> ()  [unwired: 1 in, 1 out]
      }
      frame "Scanning" {
        w576 = "%8f"  # format string
        w575 = ","  # delimiter (Tab)
        w603 = 0.0  # t0
        # "This creates time gap between subsequent\n reads in order to fill FIFO"
        n192 = xnode "Read/Write Control"("FPGA VI Reference In"=w581, "error in"=w595) -> ("FPGA VI Reference Out"=w566:refnum<k20>, "error out"=w565:errorcluster, "Number of Data Strings"=→"Number of Data Strings":i32, "FPGA state"=w560:T9)
        n193 = local read "Datalog Time Period (uSec)"() -> (w601:u32)
        n194 = Not Equal?(x=T9."Run", y=w560) -> (x != y?=w557:bool)
        n195 = Multiply(x=1e-06, y=w601) -> (x*y=w598:dbl)
        "Datalog Time Period (sec)" <- w598
        n196 = local read "Trigger Frequency (Hz)"() -> (w538:dbl)
        n197 = xnode "Invoke Method"("FPGA VI Reference In"=w566, "error in"=w565, "Number of Elements"=u32 0, "Timeout (ms)"=0) -> ("FPGA VI Reference Out"=w563:refnum<k20>, "error out"=w564:errorcluster, "Elements Remaining"=w542:u32)  [unwired: 1 out]
        n198 = Divide(x=1.0, y=w598) -> (x/y=w569:dbl)
        "Datalog Rate (Hz)" <- w569
        n199 = Multiply(x="FIFO Time Period", y=w569) -> (x*y=w539:dbl)
        n200 = Multiply(x=w539, y=5 ("Number of Data Strings 2")) -> (x*y=w567:dbl)
        n201 = To Unsigned Long Integer(number=w567) -> (unsigned 32bit integer=w562:u32)
        "Number of Elements" <- w562
        n202 = Divide(x=w538, y=w539) -> (x/y=w537:dbl)
        n203 = Divide(x=i16 1000, y=w537) -> (x/y=w535:dbl)
        n204 = Max & Min(x=w542, y=w562) -> (min(x,y)=w541:u32)  [unwired: 1 out]
        "Elements Available in FIFO" <- w541
        n205 = Equal?(x=u32 0, y=w542) -> (x = y?=w558:bool)
        n206 = And(x=w557, y=w558) -> (x .and. y?=w556:bool)
        n207 = xnode "Invoke Method"("FPGA VI Reference In"=w563, "error in"=w564, "Number of Elements"=w541, "Timeout (ms)"="Timeout (ms)") -> ("FPGA VI Reference Out"=w580:refnum<k20>, "error out"=w579:errorcluster, "Data"=w597:fxp<+/-,58,25>[], "Elements Remaining"=→"Elements Remaining" →"Elements Remaining in FIFO":u32)
        "Data" <- w597
        n208 = Decimate 1D Array(w597) -> (w552:fxp<+/-,58,25>[], w551:fxp<+/-,58,25>[], w550:fxp<+/-,58,25>[], w549:fxp<+/-,58,25>[], w582:fxp<+/-,58,25>[])
        n209 = To Quad Integer(1:w535) -> (0:w534:i64)
        n210 = Build Array(w552, w551, w550, w549, w582) -> (w604:fxp<+/-,58,25>[][])
        n211 = To Double Precision Float(number=w604) -> (double precision float=w599:dbl[][])
        n212 = Transpose 2D Array(2D array=w599) -> (transposed array=w594:dbl[][])
        n213 = case shown="True" w556 {
          tunnel: w555 -> [w609 w610]
          tunnel: [w607 w610] -> w554
          frame False {
            # "Either FIFO not empty or FPGA not \ndone running -- repeat scanning state"
            n214 = Insert Into Array(array=w609, index=0, new element=State_Enum."Scanning" ("new element/subarray")) -> (w607:T10[])
          }
          frame True {
            # "FIFO empty, FPGA done running \n-- moving onto next state"
          }
        }
        n215 = Bundle("t0"=w603, w598, w599) -> (→"Reference and Actual positions":cluster{"t0":dbl, dbl, dbl[][]})  [unwired: 1 in]
        n216 = Array To Spreadsheet String(delimiter (Tab)=w575, array=w594, 3:w576) -> (spreadsheet string=w574:string)
        n217 = call "Convert to Dynamic Data"("Array"=w552) -> ("Dynamic Data Type"=w589:dynamicdata)  [unwired: 3 in]
        n218 = call "Convert to Dynamic Data2"("Array"=w551) -> ("Dynamic Data Type"=w583:dynamicdata)  [unwired: 3 in]
        n219 = call "Convert to Dynamic Data3"("Array"=w550) -> ("Dynamic Data Type"=w585:dynamicdata)  [unwired: 3 in]
        n220 = call "Convert to Dynamic Data4"("Array"=w549) -> ("Dynamic Data Type"=w584:dynamicdata)  [unwired: 3 in]
        n221 = call "Data_Write.vi"("error initialize"=w595, "Data"=w574, "Command List"=Data_Write_Control."Write") -> ("error out"=w573:errorcluster)  [unwired: 5 in, 1 out]
        n222 = To Double Precision Float(number=w552) -> (double precision float=w548:dbl[])
        n223 = To Double Precision Float(number=w551) -> (double precision float=w547:dbl[])
        n224 = To Double Precision Float(number=w550) -> (double precision float=w546:dbl[])
        n225 = To Double Precision Float(number=w549) -> (double precision float=w545:dbl[])
        n226 = call "Convert from Dynamic Data"("Dynamic Data Type"=w589) -> ("Array"=w590:dbl[])  [unwired: 3 in]
        n227 = call "Convert from Dynamic Data2"("Dynamic Data Type"=w583) -> ("Array"=w588:dbl[])  [unwired: 3 in]
        n228 = call "Convert from Dynamic Data3"("Dynamic Data Type"=w585) -> ("Array"=w587:dbl[])  [unwired: 3 in]
        n229 = call "Convert from Dynamic Data4"("Dynamic Data Type"=w584) -> ("Array"=w586:dbl[])  [unwired: 3 in]
        n230 = Bundle(w546, w545) -> (→"XY Graph 4":cluster{dbl[], dbl[]})  [unwired: 1 in]
        n231 = Bundle(w548, w547) -> (→"XY Graph 3":cluster{dbl[], dbl[]})  [unwired: 1 in]
        n232 = Bundle("Array"=w590, "Array"=w588) -> (→"XY Ref":cluster{"Array":dbl[], "Array":dbl[]})  [unwired: 1 in]